vi "Host.vi"() -> ()   [LabVIEW 2019]
uses:
  <vilib>/Analysis/7linalg.llb/Eigenvalue and Vectors Output Option.ctl
  <vilib>/Analysis/baseanly.llb/Matrix Type of Inverse Matrix.ctl
  <vilib>/Analysis/7linalg.llb/Real Generalized Eigenvalues and Vectors.vi
  <vilib>/Analysis/7linalg.llb/Real Cholesky Factorization.vi
  <vilib>/Analysis/baseanly.llb/Full Cholesky Factorization.vi
  <vilib>/Analysis/baseanly.llb/Full Real Matrix Cholesky Factorization.vi
  <vilib>/FPGAPlugInAG/PXIe-7915/niLvFpga_Open_PXIe-7915.vi
  <vilib>/rvi/interface/common/dynamic/niFpgaDynamicAddResources.vi
  <vilib>/Analysis/baseanly.llb/Real Inverse Matrix.vi
  <vilib>/Analysis/Matrix/Numeric/Multiply/Multiply - RM,RM.vi
  <vilib>/Analysis/7linalg.llb/Real Eigenvalues and Vectors.vi
  <vilib>/Analysis/Matrix/Numeric/Add/Add - RM,RM.vi
  <vilib>/Utility/error.llb/Error Cluster From Error Code.vi
  <vilib>/rvi/errors/niLvFpgaAdjustHostInterfaceError.vi
  <vilib>/FPGAPlugInAG/Dynamic/niLvFpga_Run_Dynamic.vi
  <vilib>/FPGAPlugInAG/Dynamic/niLvFpga_Close_Dynamic.vi
  <vilib>/rvi/interface/nirviOpenFPGA/nirviOpenFPGA.xnode
  FPGA Bitfiles/choleskyfpgav1_FPGATarget_Target_pw4vIyGlOjs.lvbitx
  Target.vi
  <vilib>/rvi/interface/nirviMethod/nirviMethod.xnode
  <vilib>/rvi/interface/nirviReadWriteControl/nirviReadWriteControl.xnode
  <vilib>/rvi/interface/nirviCloseFPGA/nirviCloseFPGA.xnode
  <vilib>/Analysis/NI_AALPro.lvlib
  <vilib>/Analysis/NI_AALBase.lvlib
  <vilib>/Analysis/Matrix/NI_Matrix.lvlib
  <vilib>/rvi/errors/niLvFpgaMergeErrorWithErrorCode.vi
  <vilib>/FPGAPlugInAG/Dynamic/niLvFpga_ReadFifo_Dynamic.vi
  <vilib>/FPGAPlugInAG/Dynamic/niLvFpga_WriteFifo_Dynamic.vi
  NiFpgaLv.dll
  <vilib>/rvi/interface/Simulation/niFpgaSimulationCallBeginRW.vi
panel:
  out "T3 us":u32
  out "data output time (us)":u32
  out "data input time (us)":u32
  out "total time (us)":u32
  out "T5 ms":u32
  out "T1 us":u32
  out "data output time (ticks)":u32
  out "data input time (ticks)":u32
  out "total time (ticks)":u32
  out "T5":u32
  out "T4":u32
  out "T3":u32
  out "T2":u32
  out "T1":u32
  out "Frequencies":dbl[](array[numeric])
  out "Eigenvalues":cdb[][](array[numeric]) format="%#_4g"
  out "Run Time (ms)":u32 format="%_6f"
  out "Elements Remaining 2":u32
  out "Elements Remaining":u32
  out "K input":dbl[][](array[numeric])
  in  "Method":i32(listbox)
  out "M input":dbl[][](array[numeric])
  # "Takes 56 ms to solve without timed loop"
  # "base"
  # "1087"
  # "2174"
  # "1087"
  # "97"
  # "1087"
  # "1183"
  # "eith timed loops"
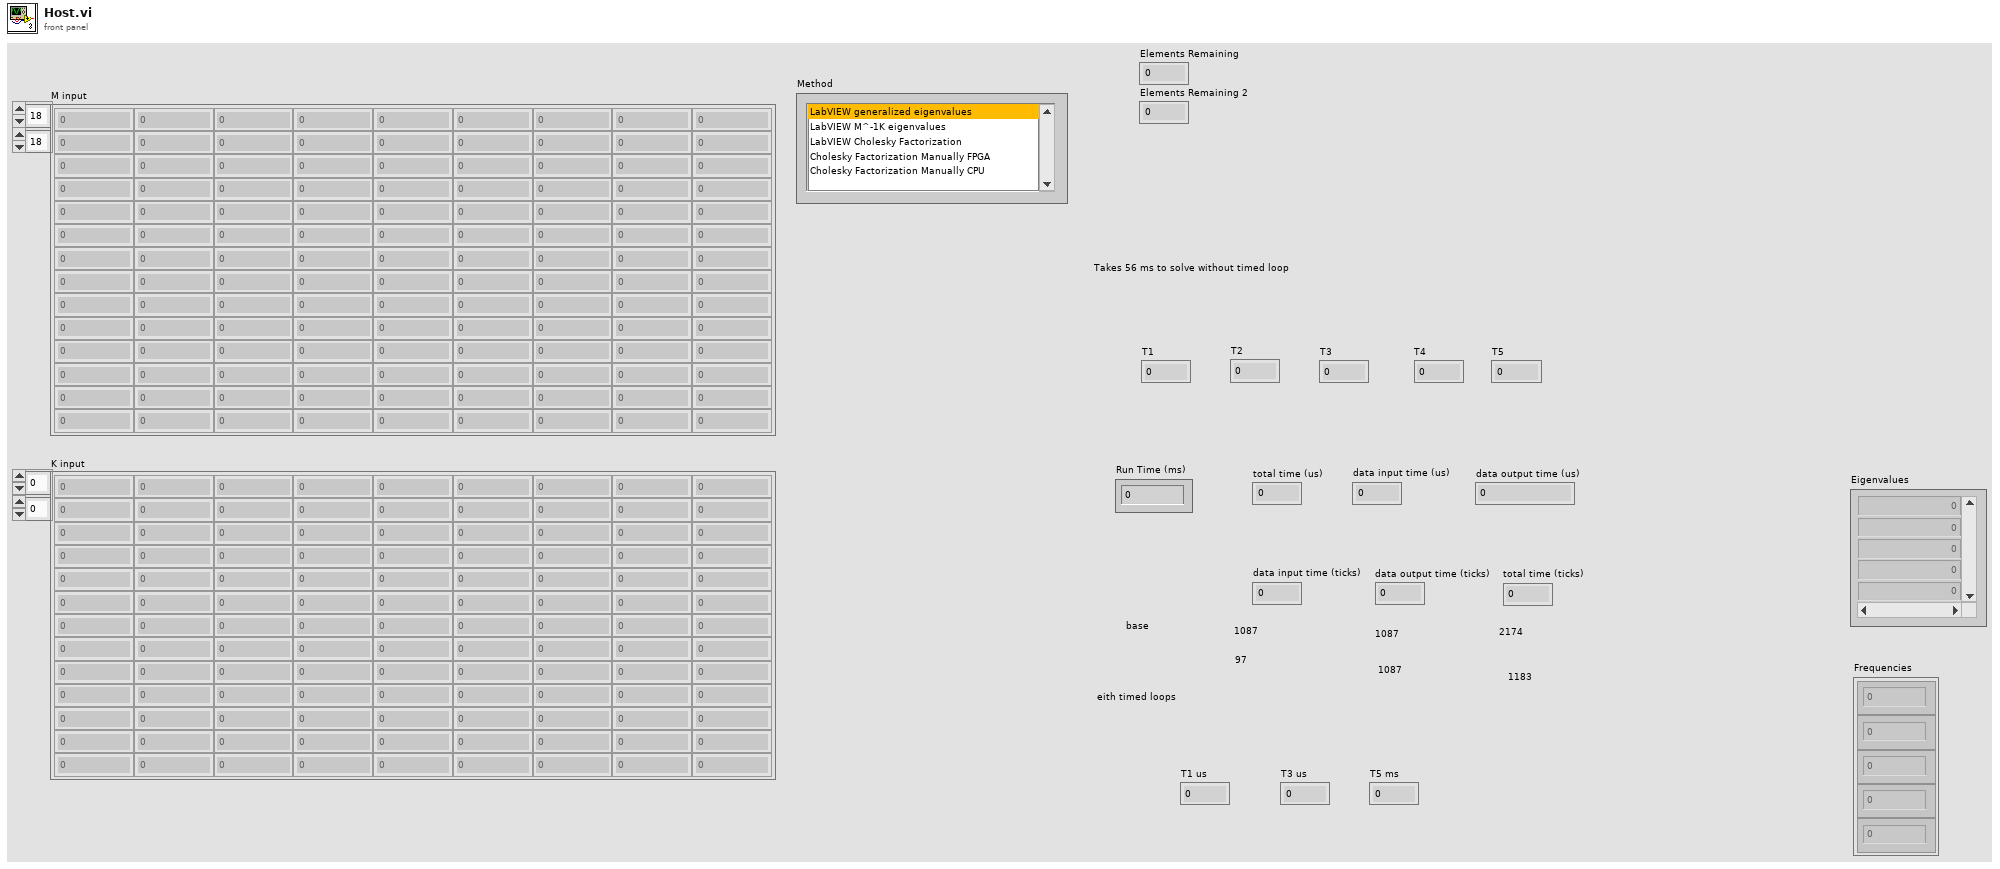
[diagram p1: front panel]
types:
  T1 = typedef "NI_AALBase.lvlib/Matrix Type of Inverse Matrix.ctl" = enum32{"General", "Positive Definite", "Lower Triangular", "Upper Triangular"}
  T2 = typedef "NI_AALPro.lvlib/Eigenvalue and Vectors Output Option.ctl" = i32
  T3 = typedef "NI_Matrix.lvlib/RealMatrix.ctl" = dbl[][]
  T4 = typedef "NI_Matrix.lvlib/ComplexMatrix.ctl" = cdb[][]
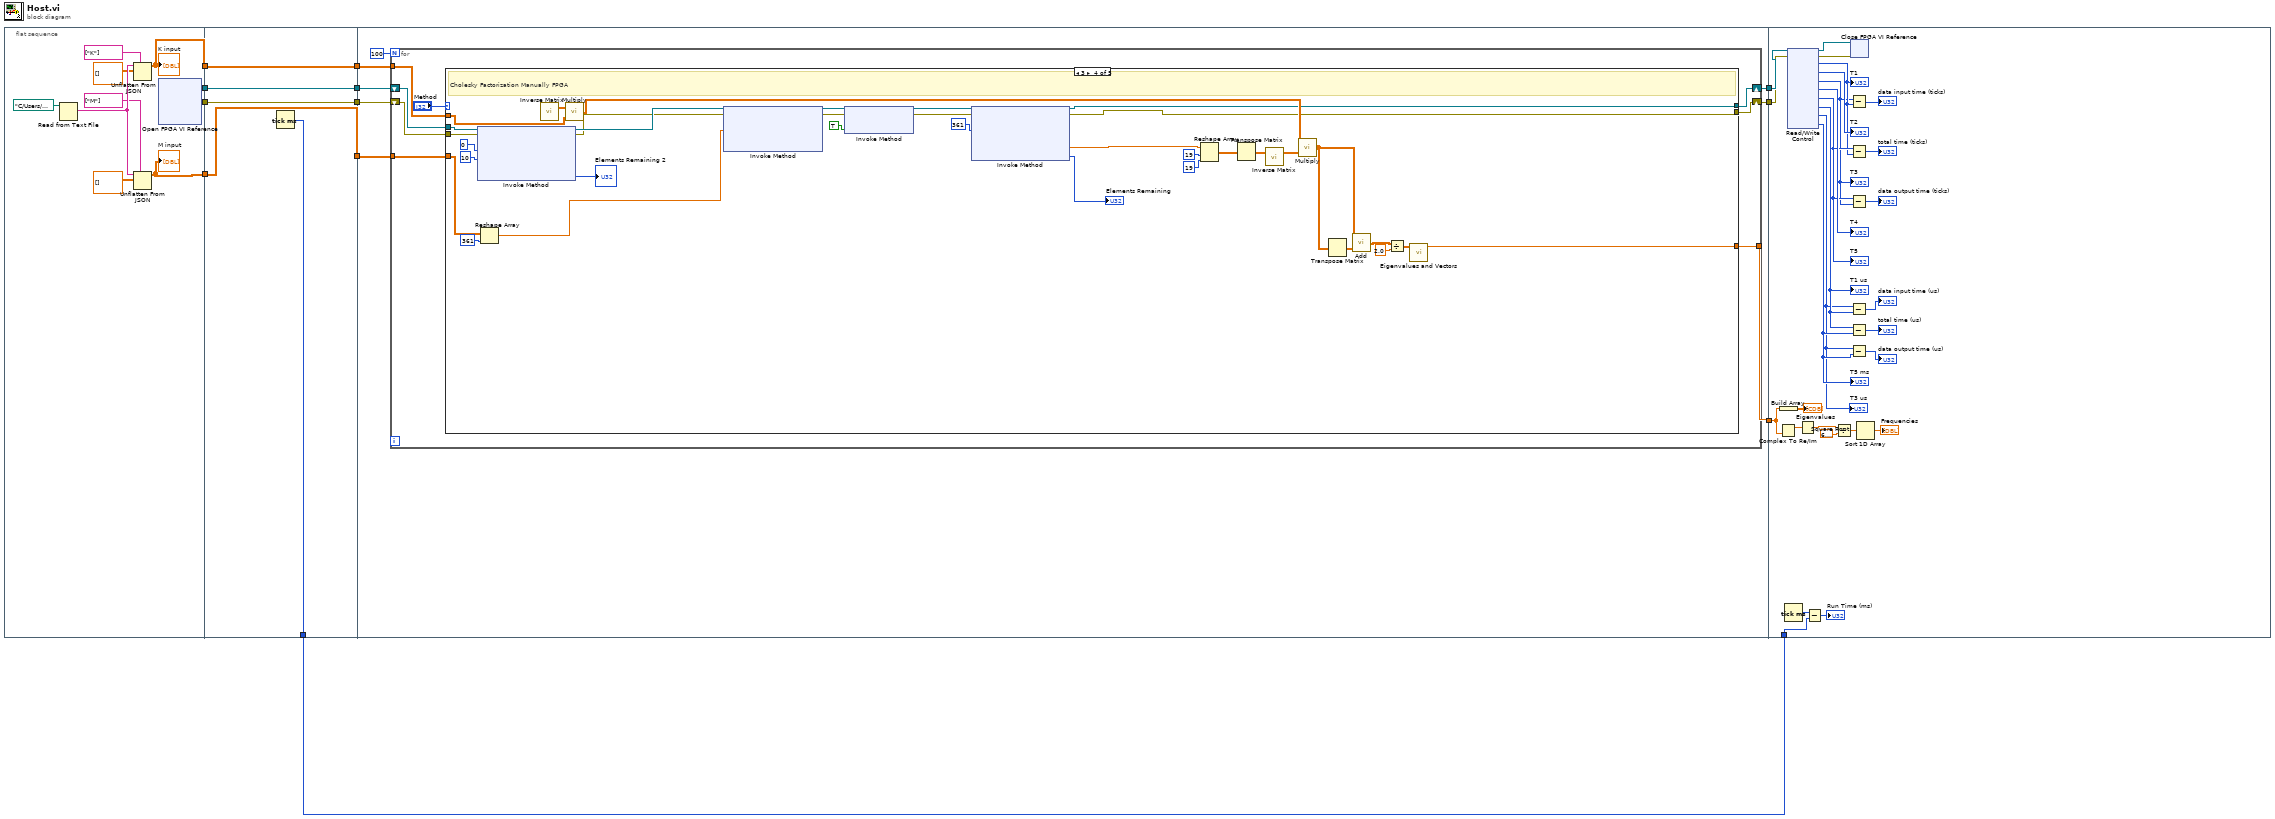
[diagram p0: block diagram]
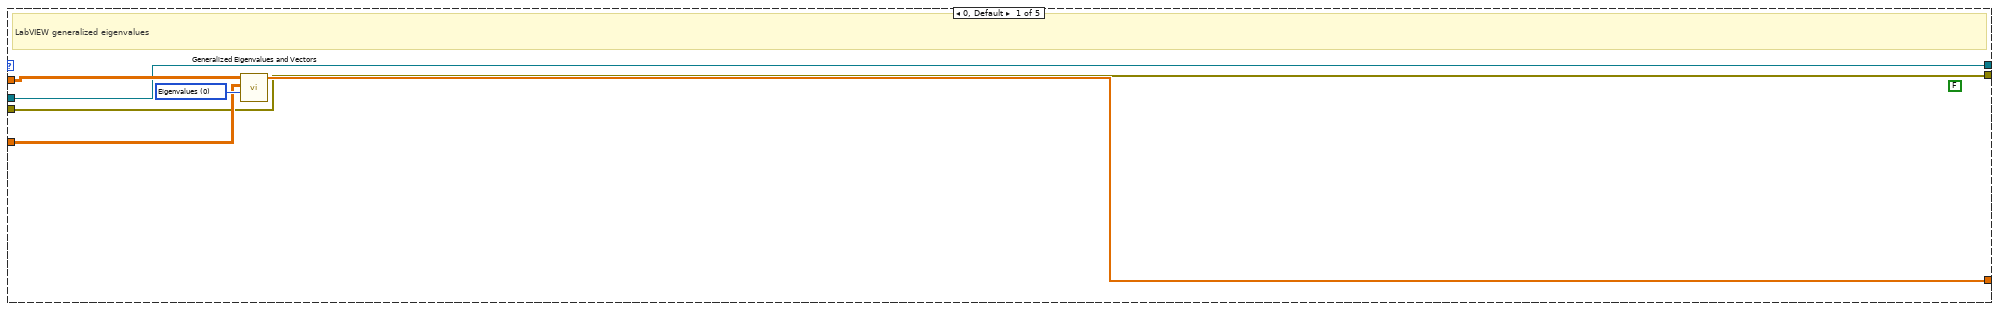
[diagram p2: hidden frame]
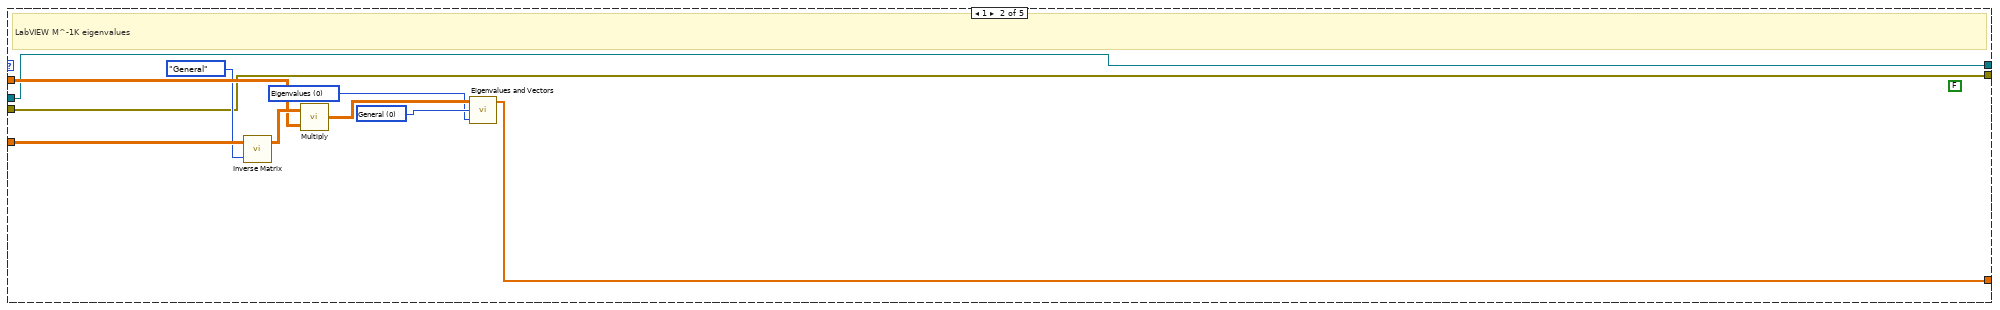
[diagram p3: hidden frame]
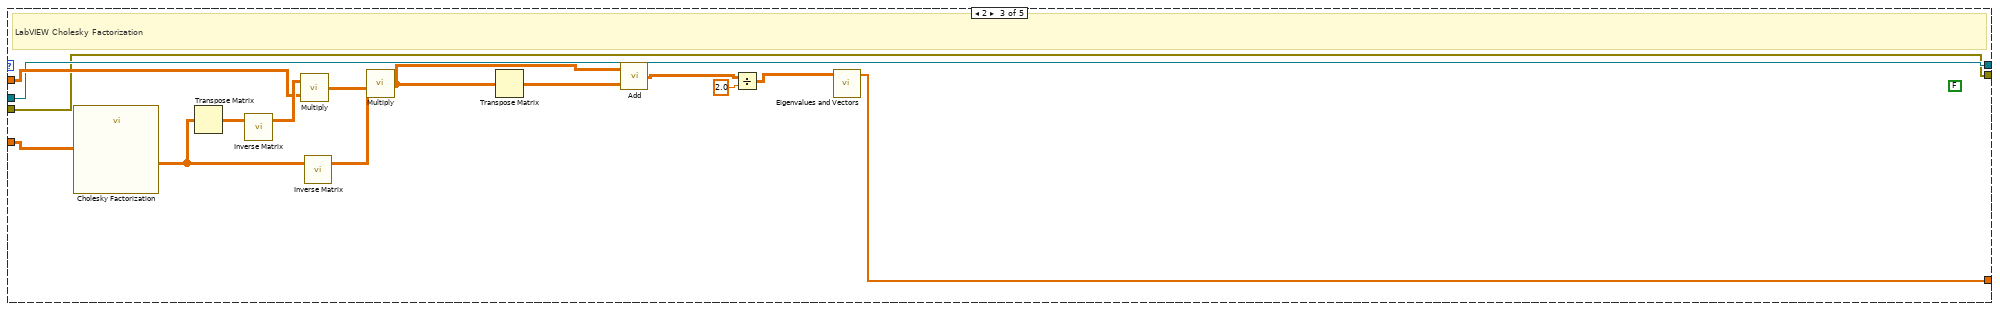
[diagram p4: hidden frame]
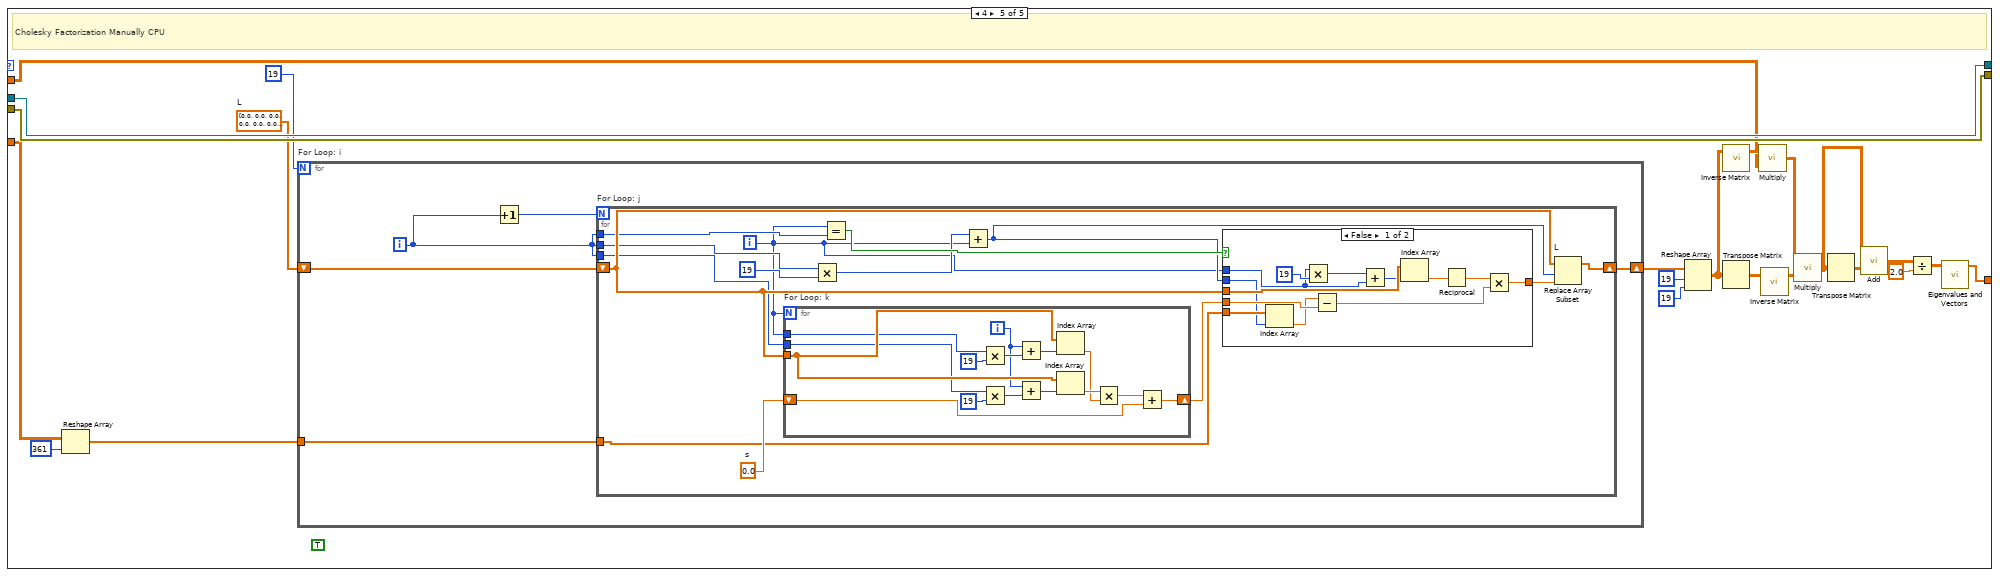
[diagram p5: hidden frame]
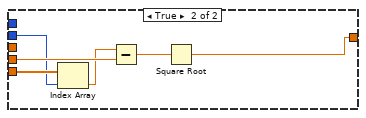
[diagram p6: hidden frame]
diagram:
  n1 = flat-sequence {
    tunnel: [w16] -> w10
    tunnel: [w15] -> w9
    tunnel: [w14] -> w7
    tunnel: [w13] -> w5
    tunnel: [w27] -> w12
    tunnel: [w26] -> w11
    tunnel: [w25] -> w1
    tunnel: w10 -> [w27]
    tunnel: w9 -> [w26]
    tunnel: [w24] -> w8
    tunnel: w7 -> [w24]
    tunnel: [w23] -> w6
    tunnel: w5 -> [w23]
    tunnel: w12 -> [w35]
    tunnel: w11 -> [w34]
    tunnel: w8 -> [w29]
    tunnel: w6 -> [w28]
    tunnel: [w33] -> w4
    tunnel: [w31] -> w3
    tunnel: [w30] -> w2
    tunnel: w4 -> [w203]
    tunnel: w3 -> [w202]
    tunnel: w2 -> [w201]
    tunnel: w1 -> [w200]
    frame #0 {
      n2 = Read from Text File(file (use dialog)=path "C:/Users/PXIe-8880/Documents/AFRL_summer_2019/Cholesky_FPGA/Cholesky_FPGA_V1/data/data.txt") -> (text=w22:string)  [unwired: 3 in, 3 out]
      n3 = Unflatten From JSON(path=string[] ["K"], JSON string=w22, type and defaults=dbl[][] []) -> (value=w15:dbl[][])  [unwired: 4 in, 1 out]
      "K input" <- w15
      n4 = Unflatten From JSON(path=string[] ["M"], JSON string=w22, type and defaults=dbl[][] []) -> (value=w16:dbl[][])  [unwired: 4 in, 1 out]
      "M input" <- w16
      n5 = xnode "Open FPGA VI Reference"() -> ("FPGA VI Reference Out"=w14:refnum<k20>, "error out"=w13:errorcluster)  [unwired: 2 in]
    }
    frame #1 {
      n6 = Tick Count (ms)() -> (millisecond timer value=w25:u32)
    }
    frame #2 {
      n7 = for {
        N: 100 -> [_]
        tunnel: w35 -> [w43]
        tunnel: w34 -> [w42]
        tunnel: [w39] -> w33
        shift-right: [w41] -> w31
        shift-left: w29 -> [w37]
        shift-right: [w40] -> w30
        shift-left: w28 -> [w36]
        n8 = case shown="3" "Method" {
          tunnel: [w48 w55 w68 w93 w109] -> w39
          tunnel: w43 -> [w47 w54 w74 w108 w110]
          tunnel: w42 -> [w46 w53 w70 w94 w111]
          tunnel: w37 -> [w45 w51 w61 w83 w130]
          tunnel: [w45 w51 w61 w87 w130] -> w41
          tunnel: w36 -> [w44 w50 w60 w82 w129]
          tunnel: [w44 w50 w60 w88 w129] -> w40
          frame 0, Default {
            (unwired) FALSE
            w49 = T2 0 items=["Eigenvalues", "Eigenvalues & Vectors"] ("output option")
            # "LabVIEW generalized eigenvalues"
            n9 = call-poly <vilib>:"Generalized Eigenvalues and Vectors.vi"("output option"=w49, "B"=w47, "A"=w46) -> ("Eigenvalues"=w48:cdb[])  [unwired: 3 in, 2 out]
          }
          frame 1 {
            (unwired) FALSE
            w56 = T2 0 items=["Eigenvalues", "Eigenvalues & Vectors"] ("output option")
            w57 = 0 items=["General", "Symmetric"] ("matrix type")
            # "LabVIEW M^-1K eigenvalues"
            n10 = call-poly <vilib>:"Inverse Matrix.vi"("matrix type"=Matrix_Type_of_Inverse_Matrix."General", "Input Matrix"=w54) -> ("Inverse Matrix"=w58:T3)  [unwired: 1 out]
            n11 = call-poly <vilib>:"Multiply.vi"("Real Matrix B"=w53, "Real Matrix A"=w58) -> ("A * B"=w59:T3)
            n12 = call-poly <vilib>:"Eigenvalues and Vectors.vi"("output option"=w56, "matrix type"=w57, "Input Matrix"=w59) -> ("Eigenvalues"=w55:cdb[])  [unwired: 2 out]
          }
          frame 2 {
            (unwired) FALSE
            # "LabVIEW Cholesky Factorization"
            n13 = call-poly <vilib>:"Cholesky Factorization.vi"("A"=w74) -> ("Cholesky"=w72:T3)  [unwired: 1 out]
            n14 = Transpose Matrix(1:w72) -> (0:w73:T3)
            n15 = call-poly <vilib>:"Inverse Matrix.vi"("Input Matrix"=w73) -> ("Inverse Matrix"=w71:T3)  [unwired: 1 in, 1 out]
            n16 = call-poly <vilib>:"Multiply.vi"("Real Matrix B"=w70, "Real Matrix A"=w71) -> ("A * B"=w67:T3)
            n17 = call-poly <vilib>:"Inverse Matrix.vi"("Input Matrix"=w72) -> ("Inverse Matrix"=w69:T3)  [unwired: 1 in, 1 out]
            n18 = call-poly <vilib>:"Multiply.vi"("Real Matrix B"=w69, "Real Matrix A"=w67) -> ("A * B"=w66:T3)
            n19 = Transpose Matrix(1:w66) -> (0:w65:T3)
            n20 = call-poly <vilib>:"Add.vi"("Real Matrix B"=w65, "Real Matrix A"=w66) -> ("A + B"=w63:T3)
            n21 = Divide(x=w63, y=2.0) -> (x/y=w62:T3)
            n22 = call-poly <vilib>:"Eigenvalues and Vectors.vi"("Input Matrix"=w62) -> ("Eigenvalues"=w68:cdb[])  [unwired: 2 in, 2 out]
          }
          frame 3 {
            # "Cholesky Factorization Manually FPGA"
            n23 = xnode "Invoke Method"("FPGA VI Reference In"=w83, "error in"=w82, "Number of Elements"=u32 0, "Timeout (ms)"=10) -> ("FPGA VI Reference Out"=w81:refnum<k20>, "error out"=w80:errorcluster, "Elements Remaining"=→"Elements Remaining 2":u32)  [unwired: 1 out]
            n24 = Reshape Array(w108, 361 ("dimension size")) -> (w76:dbl[])
            n25 = call-poly <vilib>:"Inverse Matrix.vi"() -> ("Inverse Matrix"=w103:T3)  [unwired: 2 in, 1 out]
            n26 = call-poly <vilib>:"Multiply.vi"("Real Matrix B"=w94, "Real Matrix A"=w103) -> ("A * B"=w101:T3)
            n27 = xnode "Invoke Method"("FPGA VI Reference In"=w81, "error in"=w80, "Data"=w76) -> ("FPGA VI Reference Out"=w92:refnum<k20>, "error out"=w91:errorcluster)  [unwired: 1 in, 1 out]
            n28 = xnode "Invoke Method"("FPGA VI Reference In"=w92, "error in"=w91, "Wait Until Done (F)"=TRUE) -> ("FPGA VI Reference Out"=w90:refnum<k20>, "error out"=w89:errorcluster)
            n29 = xnode "Invoke Method"("FPGA VI Reference In"=w90, "error in"=w89, "Number of Elements"=u32 361) -> ("FPGA VI Reference Out"=w87:refnum<k20>, "error out"=w88:errorcluster, "Data"=w75:sgl[], "Elements Remaining"=→"Elements Remaining":u32)  [unwired: 1 in]
            n30 = Reshape Array(w75, 19 ("dimension size"), 19 ("dimension size")) -> (w77:sgl[][])
            n31 = Transpose Matrix(1:w77) -> (0:w95:dbl[][])
            n32 = call-poly <vilib>:"Inverse Matrix.vi"("Input Matrix"=w95) -> ("Inverse Matrix"=w102:T3)  [unwired: 1 in, 1 out]
            n33 = call-poly <vilib>:"Multiply.vi"("Real Matrix B"=w102, "Real Matrix A"=w101) -> ("A * B"=w100:T3)
            n34 = Transpose Matrix(1:w100) -> (0:w99:T3)
            n35 = call-poly <vilib>:"Add.vi"("Real Matrix B"=w99, "Real Matrix A"=w100) -> ("A + B"=w97:T3)
            n36 = Divide(x=w97, y=2.0) -> (x/y=w96:T3)
            n37 = call-poly <vilib>:"Eigenvalues and Vectors.vi"("Input Matrix"=w96) -> ("Eigenvalues"=w93:cdb[])  [unwired: 2 in, 2 out]
          }
          frame 4 {
            w128 = sgl[] [0.0, 0.0, 0.0, 0.0, 0.0, 0.0, 0.0, 0.0, 0.0, 0.0, 0.0, 0.0, 0.0, 0.0, 0.0, 0.0, 0.0, 0.0, 0.0, 0.0, 0.0, 0.0, 0.0, 0.0, 0.0, 0.0, 0.0, 0.0, 0.0, 0.0, 0.0, 0.0, 0.0, 0.0, 0.0, 0.0, 0.0, 0.0, 0.0, 0.0, 0.0, 0.0, 0.0, 0.0, 0.0, 0.0, 0.0, 0.0, 0.0, 0.0, 0.0, 0.0, 0.0, 0.0, 0.0, 0.0, 0.0, 0.0, 0.0, 0.0, 0.0, 0.0, 0.0, 0.0, 0.0, 0.0, 0.0, 0.0, 0.0, 0.0, 0.0, 0.0, 0.0, 0.0, 0.0, 0.0, 0.0, 0.0, 0.0, 0.0, 0.0, 0.0, 0.0, 0.0, 0.0, 0.0, 0.0, 0.0, 0.0, 0.0, 0.0, 0.0, 0.0, 0.0, 0.0, 0.0, 0.0, 0.0, 0.0, 0.0, 0.0, 0.0, 0.0, 0.0, 0.0, 0.0, 0.0, 0.0, 0.0, 0.0, 0.0, 0.0, 0.0, 0.0, 0.0, 0.0, 0.0, 0.0, 0.0, 0.0, 0.0, 0.0, 0.0, 0.0, 0.0, 0.0, 0.0, 0.0, 0.0, 0.0, 0.0, 0.0, 0.0, 0.0, 0.0, 0.0, 0.0, 0.0, 0.0, 0.0, 0.0, 0.0, 0.0, 0.0, 0.0, 0.0, 0.0, 0.0, 0.0, 0.0, 0.0, 0.0, 0.0, 0.0, 0.0, 0.0, 0.0, 0.0, 0.0, 0.0, 0.0, 0.0, 0.0, 0.0, 0.0, 0.0, 0.0, 0.0, 0.0, 0.0, 0.0, 0.0, 0.0, 0.0, 0.0, 0.0, 0.0, 0.0, 0.0, 0.0, 0.0, 0.0, 0.0, 0.0, 0.0, 0.0, 0.0, 0.0, 0.0, 0.0, 0.0, 0.0, 0.0, 0.0, 0.0, 0.0, 0.0, 0.0, 0.0, 0.0, 0.0, 0.0, 0.0, 0.0, 0.0, 0.0, 0.0, 0.0, 0.0, 0.0, 0.0, 0.0, 0.0, 0.0, 0.0, 0.0, 0.0, 0.0, 0.0, 0.0, 0.0, 0.0, 0.0, 0.0, 0.0, 0.0, 0.0, 0.0, 0.0, 0.0, 0.0, 0.0, 0.0, 0.0, 0.0, 0.0, 0.0, 0.0, 0.0, 0.0, 0.0, 0.0, 0.0, 0.0, 0.0, 0.0, 0.0, 0.0, 0.0, 0.0, 0.0, 0.0, 0.0, 0.0, 0.0, 0.0, 0.0, 0.0, 0.0, 0.0, 0.0, 0.0, 0.0, 0.0, 0.0, 0.0, 0.0, 0.0, 0.0, 0.0, 0.0, 0.0, 0.0, 0.0, 0.0, 0.0, 0.0, 0.0, 0.0, 0.0, 0.0, 0.0, 0.0, 0.0, 0.0, 0.0, 0.0, 0.0, 0.0, 0.0, 0.0, 0.0, 0.0, 0.0, 0.0, 0.0, 0.0, 0.0, 0.0, 0.0, 0.0, 0.0, 0.0, 0.0, 0.0, 0.0, 0.0, 0.0, 0.0, 0.0, 0.0, 0.0, 0.0, 0.0, 0.0, 0.0, 0.0, 0.0, 0.0, 0.0, 0.0, 0.0, 0.0, 0.0, 0.0, 0.0, 0.0, 0.0, 0.0, 0.0, 0.0, 0.0, 0.0, 0.0, 0.0, 0.0, 0.0, 0.0, 0.0, 0.0, 0.0, 0.0, 0.0, 0.0, 0.0, 0.0, 0.0, 0.0, 0.0, 0.0, 0.0, 0.0, 0.0, 0.0, 0.0, 0.0, 0.0, 0.0, 0.0, 0.0, 0.0]  # L
            (unwired) TRUE
            # "Cholesky Factorization Manually CPU"
            n38 = Reshape Array(w110, 361 ("dimension size")) -> (w125:dbl[])
            n39 = for "For Loop: i" {
              N: 19 -> [_]
              shift-right: [w133] -> w113
              shift-left: w128 -> [w135]
              tunnel: w125 -> [w132]
              i -> [w131]
              n40 = Increment(x=w131) -> (x+1=w134:i32)
              n41 = for "For Loop: j" {
                N: w134 -> [_]
                tunnel: w131 -> [w143]
                shift-right: [w145] -> w133
                shift-left: w135 -> [w144]
                tunnel: w131 -> [w142]
                tunnel: w132 -> [w139]
                tunnel: w131 -> [w137]
                i -> [w136]
                w148 = sgl 0.0  # s
                n42 = for "For Loop: k" {
                  N: w136 -> [_]
                  tunnel: w144 -> [w182]
                  shift-right: [w178] -> w147
                  shift-left: w148 -> [w179]
                  tunnel: w137 -> [w177]
                  tunnel: w136 -> [w170]
                  i -> [w169]
                  n43 = Multiply(x=w170, y=19) -> (x*y=w172:i32)
                  n44 = Multiply(x=w177, y=19) -> (x*y=w175:i32)
                  n45 = Add(x=w169, y=w172) -> (x+y=w171:i32)
                  n46 = Add(x=w169, y=w175) -> (x+y=w174:i32)
                  n47 = Index Array(array=w182, index=w171) -> (element=w181:sgl)
                  n48 = Index Array(array=w182, index=w174) -> (element=w183:sgl)
                  n49 = Multiply(x=w183, y=w181) -> (x*y=w180:sgl)
                  n50 = Add(x=w180, y=w179) -> (x+y=w178:sgl)
                }
                n51 = Multiply(x=w142, y=19) -> (x*y=w140:i32)
                n52 = Equal?(x=w136, y=w143) -> (x = y?=w149:bool)
                n53 = Add(x=w140, y=w136) -> (x+y=w138:i32)
                n54 = case shown="False" w149 {
                  tunnel: w147 -> [w160 w168]
                  tunnel: [w159 w166] -> w146
                  tunnel: w144 -> [w162 _]
                  tunnel: w139 -> [w156 w165]
                  tunnel: w138 -> [w155 w164]
                  tunnel: w136 -> [w151 _]
                  frame False {
                    n55 = Index Array(array=w156, index=w155) -> (element=w154:dbl)
                    n56 = Multiply(x=w151, y=19) -> (x*y=w152:i32)
                    n57 = Subtract(x=w154, y=w160) -> (x-y=w157:dbl)
                    n58 = Add(x=w152, y=w151) -> (x+y=w150:i32)
                    n59 = Index Array(array=w162, index=w150) -> (element=w161:sgl)
                    n60 = Reciprocal(x=w161) -> (1/x=w158:sgl)
                    n61 = Multiply(x=w158, y=w157) -> (x*y=w159:dbl)
                  }
                  frame True {
                    n62 = Index Array(array=w165, index=w164) -> (element=w163:dbl)
                    n63 = Subtract(x=w163, y=w168) -> (x-y=w167:dbl)
                    n64 = Square Root(x=w167) -> (sqrt(x)=w166:dbl)
                  }
                }
                n65 = Replace Array Subset "L"(array=w144, new element=w146, index=w138) -> (w145:sgl[])
              }
            }
            n66 = Reshape Array(w113, 19 ("dimension size"), 19 ("dimension size")) -> (w112:sgl[][])
            n67 = call-poly <vilib>:"Inverse Matrix.vi"("Input Matrix"=w112) -> ("Inverse Matrix"=w122:T3)  [unwired: 1 in, 1 out]
            n68 = Transpose Matrix(1:w112) -> (0:w114:dbl[][])
            n69 = call-poly <vilib>:"Multiply.vi"("Real Matrix B"=w111, "Real Matrix A"=w122) -> ("A * B"=w120:T3)
            n70 = call-poly <vilib>:"Inverse Matrix.vi"("Input Matrix"=w114) -> ("Inverse Matrix"=w121:T3)  [unwired: 1 in, 1 out]
            n71 = call-poly <vilib>:"Multiply.vi"("Real Matrix B"=w121, "Real Matrix A"=w120) -> ("A * B"=w119:T3)
            n72 = Transpose Matrix(1:w119) -> (0:w118:T3)
            n73 = call-poly <vilib>:"Add.vi"("Real Matrix B"=w118, "Real Matrix A"=w119) -> ("A + B"=w116:T3)
            n74 = Divide(x=w116, y=2.0) -> (x/y=w115:T3)
            n75 = call-poly <vilib>:"Eigenvalues and Vectors.vi"("Input Matrix"=w115) -> ("Eigenvalues"=w109:cdb[])  [unwired: 2 in, 2 out]
          }
        }
      }
    }
    frame #3 {
      n76 = Build Array(w203) -> (→"Eigenvalues":T4)
      n77 = Complex To Re/Im ("Complex To Cartesian.vi")(x + iy=w203) -> (x=w209:dbl[])  [unwired: 1 out]
      n78 = Tick Count (ms)() -> (millisecond timer value=w199:u32)
      n79 = xnode "Read/Write Control"("FPGA VI Reference In"=w202, "error in"=w201) -> ("FPGA VI Reference Out"=w205:refnum<k20>, "error out"=w204:errorcluster, "T1"=w193:u32, "T2"=→"T2":u32, "T3"=w192:u32, "T4"=→"T4":u32, "T5"=w194:u32, "T1 us"=w188:u32, "T3 us"=w184:u32, "T5 us"=w185:u32)
      "T1" <- w193
      "T3" <- w192
      "T5" <- w194
      "T1 us" <- w188
      "T5 ms" <- w185
      "T3 us" <- w184
      n80 = Square Root ("Square Root.vi")(x=w209) -> (sqrt(x)=w210:dbl[])
      n81 = Subtract(x=w199, y=w200) -> (x-y=→"Run Time (ms)":u32)
      n82 = Divide(x=w210, y=6.283185307179586) -> (x/y=w211:dbl[])
      n83 = xnode "Close FPGA VI Reference"("FPGA VI Reference In"=w205, "error in"=w204) -> ()  [unwired: 1 out]
      n84 = Subtract(x=w192, y=w193) -> (x-y=→"data input time (ticks)":u32)
      n85 = Subtract(x=w194, y=w193) -> (x-y=→"total time (ticks)":u32)
      n86 = Subtract(x=w194, y=w192) -> (x-y=→"data output time (ticks)":u32)
      n87 = Subtract(x=w184, y=w188) -> (x-y=→"data input time (us)":u32)
      n88 = Subtract(x=w188, y=w185) -> (x-y=→"total time (us)":u32)
      n89 = Subtract(x=w184, y=w185) -> (x-y=→"data output time (us)":u32)
      n90 = Sort 1D Array(array=w211) -> (sorted array=→"Frequencies":dbl[])
    }
  }
